vi "UHR-Fleezers Control (host) - 12.7e.vi"() -> ()   [LabVIEW 2012] (continued)
                                n2063 = local read "Delta Fl. 1"() -> (w2984:dbl)
                                n2064 = local read "Delta Fl. 2"() -> (w2982:dbl)
                                n2065 = local read "Stop All"() -> (w2991:bool)
                                n2066 = local read "APD to Watch"() -> (w2983:bool)
                                n2067 = Select(t=w2984, s=w2983, f=w2982) -> (s? t:f=w2981:dbl)
                                n2068 = Not(x=w2993) -> (.not. x?=w2992:bool)
                                n2069 = Multiply(x=w2988, y=1000.0) -> (x*y=w2987:dbl)
                                n2070 = Negate(x=w2987) -> (-x=w2986:dbl)
                                n2071 = Less?(x=w2981, y=w2986) -> (x < y?=w2990:bool)
                                n2072 = Compound Arithmetic op=OR(w2990, w2991, w2992, "Reset Force") -> (w2980:bool)
                                n2073 = case shown="True" w2980 {
                                tunnel: w2997 -> [_ w3012]
                                tunnel: w2996 -> [_ w3011]
                                tunnel: w2995 -> [_ w3001]
                                tunnel: w2994 -> [_ w3003]
                                frame False {
                                }
                                frame True {
                                n2074 = local read "Time (s)"() -> (w3002:dbl)
                                n2075 = case shown="\"Yank\"" w3011 {
                                tunnel: w3012 -> [_ w3015]
                                tunnel: w3003 -> [_ w3013]
                                frame "Image", Default {
                                }
                                frame "Yank" {
                                n2076 = flat-sequence {
                                tunnel: [w3021] -> w3016
                                tunnel: w3015 -> [w3021]
                                tunnel: [w3017] -> w3014
                                tunnel: w3013 -> [w3017]
                                tunnel: w3016 -> [w3024]
                                tunnel: w3014 -> [w3022]
                                frame #0 {
                                n2077 = local read "Yank Delay (s)"() -> (w3020:dbl)
                                n2078 = Multiply(x=w3020, y=1000.0) -> (x*y=w3018:dbl)
                                n2079 = Wait (ms)(milliseconds to wait=w3018) -> ()  [unwired: 1 out]
                                }
                                frame #1 {
                                n2080 = local read "Yank to which?"() -> (w3023:bool)
                                n2081 = case shown="False" w3023 {
                                tunnel: w3024 -> [_ w3051]
                                tunnel: w3022 -> [w3025 _]
                                frame False {
                                n2082 = flat-sequence {
                                tunnel: w3025 -> [w3026]
                                frame #0 {
                                n2083 = property on="Trap Pos FB SP" class="DigNum (strict)"("Val(Sgnl)"=w3026) -> ()  [unwired: 2 in, 2 out]
                                }
                                frame #1 {
                                n2084 = Wait (ms)(milliseconds to wait=u32 700) -> ()  [unwired: 1 out]
                                }
                                frame #2 {
                                n2085 = local read "Action (%)"() -> (w3031:dbl)
                                n2086 = Absolute Value(x=w3031) -> (abs(x)=w3030:dbl)
                                n2087 = Greater?(x=w3030, y=70.0) -> (0:w3028:bool)
                                n2088 = property on="Remove Action Offset" class="Bool (strict)"("Val(Sgnl)"=w3028) -> ()  [unwired: 2 in, 2 out]
                                }
                                frame #3 {
                                n2089 = for {
                                N: 4 -> [_]
                                n2090 = flat-sequence {
                                frame #0 {
                                n2091 = Wait (ms)(milliseconds to wait=u32 500) -> ()  [unwired: 1 out]
                                }
                                frame #1 {
                                n2092 = local read "Action (%)"() -> (w3037:dbl)
                                n2093 = Absolute Value(x=w3037) -> (abs(x)=w3036:dbl)
                                n2094 = Greater?(x=w3036, y=70.0) -> (0:w3034:bool)
                                n2095 = property on="Remove Action Offset" class="Bool (strict)"("Val(Sgnl)"=w3034) -> ()  [unwired: 2 in, 2 out]
                                }
                                }
                                }
                                }
                                frame #4 {
                                n2096 = local read "Shift confocal"() -> (w3042:bool)
                                n2097 = local read "Mean"() -> (w3044:dbl)
                                n2098 = Greater?(x=w3044, y=11.0) -> (0:w3041:bool)
                                n2099 = Not(x=w3041) -> (.not. x?=w3040:bool)
                                n2100 = And(x=w3041, y=w3042) -> (x .and. y?=w3039:bool)
                                n2101 = And(x=w3040, y=w3042) -> (x .and. y?=w3038:bool)
                                n2102 = case shown="True" w3039 {
                                frame False {
                                }
                                frame True {
                                n2103 = local read "Confocal Y 2 (V)"() -> (w3048:dbl)
                                n2104 = local read "Confocal X 2 (V)"() -> (w3047:dbl)
                                n2105 = property on="AO2" class="Slide (strict)"("Val(Sgnl)"=w3047) -> ()  [unwired: 2 in, 2 out]
                                n2106 = property on="AO1" class="Slide (strict)"("Val(Sgnl)"=w3048) -> ()  [unwired: 2 in, 2 out]
                                }
                                }
                                n2107 = case shown="True" w3038 {
                                frame False {
                                }
                                frame True {
                                n2108 = local read "Confocal X 1 (V)"() -> (w3045:dbl)
                                n2109 = local read "Confocal Y 1 (V)"() -> (w3046:dbl)
                                n2110 = property on="AO1" class="Slide (strict)"("Val(Sgnl)"=w3046) -> ()  [unwired: 2 in, 2 out]
                                n2111 = property on="AO2" class="Slide (strict)"("Val(Sgnl)"=w3045) -> ()  [unwired: 2 in, 2 out]
                                }
                                }
                                }
                                frame #5 {
                                n2112 = Wait (ms)(milliseconds to wait=u32 1500) -> ()  [unwired: 1 out]
                                }
                                frame #6 {
                                n2113 = property on="Rem fb disp offset" class="Bool (strict)"("Val(Sgnl)"=TRUE ("Value (Signaling)")) -> ()  [unwired: 2 in, 2 out]
                                }
                                }
                                }
                                frame True {
                                n2114 = flat-sequence {
                                tunnel: w3051 -> [w3052]
                                frame #0 {
                                n2115 = property on="Trap Delta (MHz)" class="DigNum (strict)"("Val(Sgnl)"=w3052) -> ()  [unwired: 2 in, 2 out]
                                }
                                frame #1 {
                                n2116 = Wait (ms)(milliseconds to wait=u32 500) -> ()  [unwired: 1 out]
                                }
                                frame #2 {
                                n2117 = local read "Shift confocal"() -> (w3058:bool)
                                n2118 = local read "Mean"() -> (w3060:dbl)
                                n2119 = Greater?(x=w3060, y=11.0) -> (0:w3057:bool)
                                n2120 = Not(x=w3057) -> (.not. x?=w3056:bool)
                                n2121 = And(x=w3057, y=w3058) -> (x .and. y?=w3055:bool)
                                n2122 = And(x=w3056, y=w3058) -> (x .and. y?=w3054:bool)
                                n2123 = case shown="True" w3055 {
                                frame False {
                                }
                                frame True {
                                n2124 = local read "Confocal Y 2 (V)"() -> (w3064:dbl)
                                n2125 = local read "Confocal X 2 (V)"() -> (w3063:dbl)
                                n2126 = property on="AO2" class="Slide (strict)"("Val(Sgnl)"=w3063) -> ()  [unwired: 2 in, 2 out]
                                n2127 = property on="AO1" class="Slide (strict)"("Val(Sgnl)"=w3064) -> ()  [unwired: 2 in, 2 out]
                                }
                                }
                                n2128 = case shown="True" w3054 {
                                frame False {
                                }
                                frame True {
                                n2129 = local read "Confocal Y 1 (V)"() -> (w3062:dbl)
                                n2130 = local read "Confocal X 1 (V)"() -> (w3061:dbl)
                                n2131 = property on="AO2" class="Slide (strict)"("Val(Sgnl)"=w3061) -> ()  [unwired: 2 in, 2 out]
                                n2132 = property on="AO1" class="Slide (strict)"("Val(Sgnl)"=w3062) -> ()  [unwired: 2 in, 2 out]
                                }
                                }
                                }
                                }
                                }
                                }
                                }
                                }
                                }
                                }
                                n2133 = local read "Messages"() -> (w3010:string)
                                n2134 = Subtract(x=w3002, y=w3001) -> (x-y=w3008:dbl)
                                "Duration (s)" <- w3008
                                n2135 = Number To Decimal String(number=w3008, width (-)=i16 0) -> (decimal integer string=w3006:string)
                                n2136 = Concatenate Strings(w3006, " s fluorescence event." ("string")) -> (w3004:string)
                                n2137 = call "Update messages.vi"("Message to add"=w3004, "Old message string"=w3010) -> ("New message string"=w3009:string)
                                n2138 = local write "Reset Force"(FALSE ("Reset Force")) -> ()
                                n2139 = local write "Waiting"(TRUE ("Waiting")) -> ()
                                n2140 = local write "Messages"(w3009) -> ()
                                n2141 = local write "Fl. High"(FALSE ("Fl. High")) -> ()
                                n2142 = call <vilib>:"Beep.vi"() -> ()  [unwired: 3 in, 9 out]
                                }
                                }
                                n2143 = node-c288() -> ()  [unwired: 2 out]
                              }
                              n2144 = node-c288(w2978) -> ()  [unwired: 1 out]
                            }
                          }
                        }
                      }
                      n2145 = local read "Trap Delta (MHz)"() -> (w2893:dbl)
                      n2146 = local read "Trap Pos FB SP"() -> (w2888:fxp<+/-,16,1>)
                    }
                  }
                }
                frame #1 {
                  n2147 = local read "Stop All"() -> (w3074:bool)
                  n2148 = local read "Fl. Triggered..."() -> (w3072:bool)
                  n2149 = Not(x=w3072) -> (.not. x?=w3073:bool)
                  n2150 = Or(x=w3073, y=w3074) -> (x .or. y?=w3071:bool)
                }
              }
              n2151 = case shown="True" w2665 {
                frame False {
                }
                frame True {
                  n2152 = local read "Confocal Y 1 (V)"() -> (w2675:dbl)
                  n2153 = local read "Confocal X 1 (V)"() -> (w2674:dbl)
                  n2154 = property on="AO2" class="Slide (strict)"("Val(Sgnl)"=w2674) -> ()  [unwired: 2 in, 2 out]
                  n2155 = property on="AO1" class="Slide (strict)"("Val(Sgnl)"=w2675) -> ()  [unwired: 2 in, 2 out]
                }
              }
              n2156 = case shown="True" w2665 {
                frame False {
                }
                frame True {
                  w2673 = FALSE ("Fl. High")
                  n2157 = local write "Waiting"(w2673) -> ()
                  n2158 = local write "Fl. High"(w2673) -> ()
                }
              }
              n2159 = node-c288() -> ()  [unwired: 2 out]
            }
            n2160 = node-c288(w2663) -> ()  [unwired: 1 out]
          }
        }
      }
      event "Stop All": Value Change {
        n2161 = event-data() -> ()  [unwired: 7 out]
        n2162 = local read "Stop All"() -> (w3079:bool)
      }
    }
    n2163 = node-c288() -> ()  [unwired: 2 out]
  }
  n2164 = timed-loop "Mouse control: trap position (AOM deflection), set confocal spot from image" {
    tunnel: [w3081] -> w74
    timing: w68 -> [_]
    timing-out: [_] -> w67
    tunnel: w5 -> [w3080]
    stop <- w3081 stop-if-true
    n2165 = node-c288() -> ()  [unwired: 2 out]
    n2166 = event shown="[0] \"Pane\": Mouse Down" {
      selector: _ -> [_ _]
      dyn-events: _ -> [_ _]
      timeout: _ -> [_ _]
      tunnel: w3080 -> [w3084 _]
      event Mouse Down {
        n2167 = event-data() -> ("Time"=w3086:u32, "Coords"=w3085:T7, "Button"=w3087:u16)  [unwired: 6 out]
        n2168 = case shown="3" w3087 {
          tunnel: w3086 -> [_ _ w3193]
          tunnel: w3085 -> [_ w3124 w3191]
          tunnel: w3084 -> [_ _ w3187]
          frame 0, Default {
          }
          frame 1 {
            n2169 = property on="APD 2" class="ImageControl"() -> ("Displayed Image Position"=w3094:cluster{"Left":i32, "Top":i32})  [unwired: 2 in, 2 out]
            n2170 = property on="APD 1" class="ImageControl"() -> ("Displayed Image Position"=w3123:cluster{"Left":i32, "Top":i32})  [unwired: 2 in, 2 out]
            n2171 = property on="Detection Laser X" class="ImageControl"() -> ("Displayed Image Position"=w3120:cluster{"Left":i32, "Top":i32})  [unwired: 2 in, 2 out]
            n2172 = property on="Detection Laser Y" class="ImageControl"() -> ("Displayed Image Position"=w3119:cluster{"Left":i32, "Top":i32})  [unwired: 2 in, 2 out]
            n2173 = property on="APD 2" class="ImageControl"() -> ("Displayed Image Size"=w3093:cluster{"Width":u32, "Height":u32})  [unwired: 2 in, 2 out]
            n2174 = property on="APD 1" class="ImageControl"() -> ("Displayed Image Size"=w3121:cluster{"Width":u32, "Height":u32})  [unwired: 2 in, 2 out]
            n2175 = property on="Detection Laser X" class="ImageControl"() -> ("Displayed Image Size"=w3122:cluster{"Width":u32, "Height":u32})  [unwired: 2 in, 2 out]
            n2176 = property on="Detection Laser Y" class="ImageControl"() -> ("Displayed Image Size"=w3118:cluster{"Width":u32, "Height":u32})  [unwired: 2 in, 2 out]
            n2177 = Unbundle By Name(w3093) -> ("Width"=w3090:u32, "Height"=w3089:u32)
            n2178 = Unbundle By Name(w3094) -> ("Left"=w3092:i32, "Top"=w3091:i32)
            n2179 = Unbundle By Name(w3121) -> ("Width"=w3115:u32, "Height"=w3114:u32)
            n2180 = Unbundle By Name(w3122) -> ("Width"=w3111:u32, "Height"=w3110:u32)
            n2181 = Unbundle By Name(w3118) -> ("Width"=w3107:u32, "Height"=w3106:u32)
            n2182 = Unbundle By Name(w3123) -> ("Left"=w3117:i32, "Top"=w3116:i32)
            n2183 = Unbundle By Name(w3120) -> ("Left"=w3113:i32, "Top"=w3112:i32)
            n2184 = Unbundle By Name(w3119) -> ("Left"=w3109:i32, "Top"=w3108:i32)
            n2185 = Bundle("Left"=w3092, "Top"=w3091, "Width"=w3090, "Height"=w3089) -> (w3088:T33)  [unwired: 1 in]
            n2186 = Bundle("Left"=w3117, "Top"=w3116, "Width"=w3115, "Height"=w3114) -> (w3105:T33)  [unwired: 1 in]
            n2187 = Bundle("Left"=w3113, "Top"=w3112, "Width"=w3111, "Height"=w3110) -> (w3104:T33)  [unwired: 1 in]
            n2188 = Bundle("Left"=w3109, "Top"=w3108, "Width"=w3107, "Height"=w3106) -> (w3103:T33)  [unwired: 1 in]
            n2189 = Build Cluster Array(w3088, w3105, w3104, w3103) -> (w3102:T34)
            n2190 = for {
              tunnel: w3124 -> [w3135]
              tunnel: w3102 -> [w3136] mode=indexing
              shift-right: [w3133] -> w3100
              shift-left: TRUE -> [w3134]
              shift-right: [w3132] -> w3098
              shift-left: _ -> [w3128]
              shift-right: [w3131] -> w3097
              shift-left: _ -> [w3127]
              shift-right: [w3130] -> w3096
              shift-left: _ -> [w3126]
              shift-right: [w3129] -> w3095
              shift-left: _ -> [w3125]
              n2191 = case shown="True" w3134 {
                selector: w3134 -> [w3141 _]
                tunnel: w3136 -> [_ w3150]
                tunnel: w3135 -> [_ w3148]
                tunnel: [w3141 w3146] -> w3133
                tunnel: [w3140 w3145] -> w3132
                tunnel: [w3139 w3144] -> w3131
                tunnel: [w3138 w3143] -> w3130
                tunnel: [w3137 w3142] -> w3129
                tunnel: w3128 -> [w3140 _]
                tunnel: w3127 -> [w3139 _]
                tunnel: w3126 -> [w3138 _]
                tunnel: w3125 -> [w3137 _]
                frame False {
                }
                frame True {
                  n2192 = Unbundle(w3150) -> (w3149:T33)
                  n2193 = call "isclickinwindow.vi"("Image Param"=w3149, "Point32"=w3148) -> ("4 Y"=w3142:i32, "3 Height"=w3143:i32, "2 X"=w3144:i32, "1 Width"=w3145:i32, "In image?"=w3147:bool)  [unwired: 1 in]
                  n2194 = Not(x=w3147) -> (.not. x?=w3146:bool)
                }
              }
            }
            n2195 = Not(x=w3100) -> (.not. x?=w3099:bool)
            n2196 = case shown="True" w3099 {
              tunnel: w3097 -> [_ w3164]
              tunnel: w3095 -> [_ w3163]
              tunnel: w3098 -> [_ w3162]
              tunnel: w3096 -> [_ w3161]
              frame False {
              }
              frame True {
                w3151 = FALSE ("Get Point")
                n2197 = local read "Scan lines (y)"() -> (w3166:u64)
                n2198 = disable-structure shown="Disabled" {
                  frame Disabled {
                  }
                  frame Enabled {
                  }
                }
                n2199 = local read "Actual MCL Inc (V)"() -> (w3160:dbl)
                n2200 = local read "Scan steps (MCL)"() -> (w3165:u64)
                n2201 = Divide "Y Pix/step"(x=w3161, y=w3166) -> (x/y=w3173:dbl)
                n2202 = Divide "Y V/pix"(x=w3160, y=w3173) -> (x/y=w3172:dbl)
                n2203 = Divide "Y half step offset"(x=w3160, y=2.0) -> (x/y=w3174:dbl)
                n2204 = Divide "X pix/step"(x=w3162, y=w3165) -> (x/y=w3171:dbl)
                n2205 = Negate(x=w3174) -> (-x=w3175:dbl)
                n2206 = local read "Initial Y"() -> (w3181:dbl)
                n2207 = Multiply(x=w3163, y=w3172) -> (x*y=w3182:dbl)
                n2208 = Divide "X half step offset"(x=w3160, y=2.0) -> (x/y=w3168:dbl)
                n2209 = Divide "X V/pix"(x=w3160, y=w3171) -> (x/y=w3170:dbl)
                n2210 = Multiply(x=w3160, y=w3165) -> (x*y=w3177:dbl)
                n2211 = Compound Arithmetic op=ADD(w3175, w3182, w3181) -> (w3152:dbl)
                "Pointer Y (V)" <- w3152
                n2212 = Multiply(x=w3170, y=w3164) -> (x*y=w3179:dbl)
                n2213 = Negate(x=w3168) -> (-x=w3167:dbl)
                n2214 = local read "Initial X"() -> (w3180:dbl)
                n2215 = Negate(x=w3179) -> (-x=w3178:dbl)
                n2216 = Compound Arithmetic op=ADD(w3167, w3177, w3180, w3178) -> (w3153:dbl)
                "Pointer X (V)" <- w3153
                n2217 = case shown="True" "Set High F Confocal Spot (X-Y)" {
                  tunnel: w3153 -> [_ w3183]
                  tunnel: w3152 -> [_ w3184]
                  frame False {
                  }
                  frame True {
                    "Confocal Y 2 (V)" <- w3184
                    "Confocal X 2 (V)" <- w3183
                  }
                }
                n2218 = Or(x="Set X Only", y="Set Confocal Spot (X-Y)") -> (x .or. y?=w3156:bool)
                n2219 = Or(x="Set Confocal Spot (X-Y)", y="Set Y Only") -> (x .or. y?=w3155:bool)
                n2220 = case shown="True" w3156 {
                  tunnel: w3153 -> [_ w3185]
                  frame False {
                  }
                  frame True {
                    n2221 = property on="AO2" class="Slide (strict)"("Val(Sgnl)"=w3185) -> ()  [unwired: 2 in, 2 out]
                    "Confocal X 1 (V)" <- w3185
                  }
                }
                n2222 = case shown="True" w3155 {
                  tunnel: w3152 -> [_ w3186]
                  frame False {
                  }
                  frame True {
                    n2223 = property on="AO1" class="Slide (strict)"("Val(Sgnl)"=w3186) -> ()  [unwired: 2 in, 2 out]
                    "Confocal Y 1 (V)" <- w3186
                  }
                }
                n2224 = local write "Set High F Confocal Spot (X-Y)"(w3151) -> ()
                n2225 = local write "Set Confocal Spot (X-Y)"(w3151) -> ()
                n2226 = local write "Set X Only"(w3151) -> ()
                n2227 = local write "Set Y Only"(w3151) -> ()
              }
            }
          }
          frame 3 {
            n2228 = local read "BD 2 Frequency 1 (MHz)"() -> (w3188:dbl)
            n2229 = local read "BD 1 Frequency 1 (MHz)"() -> (w3189:dbl)
            n2230 = local write "Manipulating Trap"(TRUE ("Manipulating Trap")) -> ()
            n2231 = local write "Coords"(T7 {"Horizontal"=0, "Vertical"=0} ("Coords")) -> ()
            n2232 = while {
              tunnel: w3193 -> [w3198]
              tunnel: w3191 -> [w3197]
              tunnel: w3189 -> [w3196]
              tunnel: w3188 -> [w3195]
              tunnel: w3187 -> [w3194]
              stop <- w3199 stop-if-true
              n2233 = event shown="[0] \"Pane\": Mouse Move" {
                selector: _ -> [_ _]
                dyn-events: _ -> [_ _]
                timeout: _ -> [_ _]
                tunnel: ["Force Manip Abort" w3263] -> w3199
                tunnel: w3198 -> [w3206 _]
                tunnel: w3197 -> [w3204 _]
                tunnel: w3196 -> [w3203 _]
                tunnel: w3195 -> [w3202 _]
                tunnel: w3194 -> [w3200 _]
                event Mouse Move {
                  n2234 = event-data() -> ("Time"=w3207:u32, "Coords"=w3208:T7)  [unwired: 3 out]
                  n2235 = Less?(x=w3207, y=w3206) -> (x < y?=w3205:bool)
                  n2236 = case "Makes sure old motion events prior to mouse click aren't used" shown="False" w3205 {
                    tunnel: w3208 -> [w3250 _]
                    tunnel: w3204 -> [w3251 _]
                    tunnel: w3203 -> [w3225 _]
                    tunnel: w3202 -> [w3224 _]
                    tunnel: w3200 -> [w3209 _]
                    frame False {
                      n2237 = Subtract(x=w3250, y=w3251) -> (x-y=w3249:T7)
                      "Coords" <- w3249
                      n2238 = local read "Y RF Frequency Limits (MHz)"() -> (w3210:T16)
                      n2239 = To Double Precision Float(number=w3249) -> (double precision float=w3248:cluster{"Horizontal":dbl, "Vertical":dbl})
                      n2240 = Multiply(x=cluster{"Horizontal":dbl, "Vertical":dbl} {"Horizontal"=-1.0, "Vertical"=1.0}, y="Manipulation Scaling") -> (x*y=w3244:cluster{"Horizontal":dbl, "Vertical":dbl})
                      n2241 = local read "X RF Frequency Limits (MHz)"() -> (w3211:T16)
                      n2242 = Multiply(x=w3248, y=w3244) -> (x*y=w3246:cluster{"Horizontal":dbl, "Vertical":dbl})
                      n2243 = Unbundle By Name(w3246) -> ("Horizontal"=w3241:dbl, "Vertical"=w3245:dbl)
                      n2244 = Unbundle By Name(w3210) -> ("Maximum"=w3213:dbl, "Minimum"=w3212:dbl)
                      n2245 = Boolean To (0,1)(Boolean="Manip. X?") -> (0, 1=w3239:i16)
                      n2246 = Boolean To (0,1)(Boolean="Manip. Y?") -> (0, 1=w3236:i16)
                      n2247 = local read "BD 1 Frequency 2 (MHz)"() -> (w3227:dbl)
                      n2248 = Multiply(x=w3245, y=w3236) -> (x*y=w3238:dbl)
                      n2249 = Multiply(x=w3239, y=w3241) -> (x*y=w3242:dbl)
                      n2250 = local read "BD 2 Frequency 2 (MHz)"() -> (w3226:dbl)
                      n2251 = Unbundle By Name(w3211) -> ("Maximum"=w3215:dbl, "Minimum"=w3214:dbl)
                      n2252 = Add(x=w3224, y=w3238) -> (x+y=w3217:dbl)
                      n2253 = Add(x=w3225, y=w3242) -> (x+y=w3219:dbl)
                      n2254 = In Range and Coerce(upper limit=w3215, x=w3219, lower limit=w3214) -> (coerced(x)=w3218:dbl)  [unwired: 1 out]
                      n2255 = In Range and Coerce(upper limit=w3213, x=w3217, lower limit=w3212) -> (coerced(x)=w3216:dbl)  [unwired: 1 out]
                      n2256 = Subtract(x=w3218, y=w3227) -> (x-y=w3235:dbl)
                      n2257 = Subtract(x=w3216, y=w3226) -> (x-y=w3234:dbl)
                      n2258 = Square(x=w3235) -> (x^2=w3233:dbl)
                      n2259 = Square(x=w3234) -> (x^2=w3232:dbl)
                      n2260 = Add(x=w3233, y=w3232) -> (x+y=w3231:dbl)
                      n2261 = Square Root(x=w3231) -> (sqrt(x)=w3228:dbl)
                      n2262 = In Range and Coerce(upper limit="Limit Max (MHz)", x=w3228, lower limit="Limit Min (MHz)") -> (In Range?=w3221:bool)  [unwired: 1 out]
                      n2263 = Not(x="Limits Enable") -> (.not. x?=w3220:bool)
                      n2264 = Or(x=w3221, y=w3220) -> (x .or. y?=w3222:bool)
                      n2265 = case shown="True" w3222 {
                        tunnel: w3228 -> [_ w3253]
                        tunnel: w3218 -> [_ w3260]
                        tunnel: w3227 -> [_ w3259]
                        tunnel: w3216 -> [_ w3258]
                        tunnel: w3226 -> [_ w3257]
                        tunnel: w3211 -> [_ w3255]
                        tunnel: w3210 -> [_ w3254]
                        tunnel: w3209 -> [_ w3252]
                        frame False {
                        }
                        frame True {
                          n2266 = local read "BD 1 Frequency 3 (MHz)"() -> (w3261:dbl)
                          n2267 = local read "BD 2 Frequency 3 (MHz)"() -> (w3256:dbl)
                          n2268 = local write "Trap Delta (MHz)"(w3253) -> ()
                          n2269 = call "set RF board frequency - interlace.vi"("Board 2 Frequency Limits"=w3254, "Board 1 Frequency Limits"=w3255, "FPGA VI Reference In"=w3252, "Board 2 Frequency 3 (MHz)"=w3256, "Board 1 Frequency 3 (MHz)"=w3261, "Board 2 Frequency 2 (MHz)"=w3257, "Board 2 Frequency 1 (MHz)"=w3258, "Board 1 Frequency 2 (MHz)"=w3259, "Board 1 Frequency 1  (MHz)"=w3260) -> ()  [unwired: 1 in, 2 out]
                          n2270 = local write "BD 2 Frequency 1 (MHz)"(w3258) -> ()
                          n2271 = local write "BD 1 Frequency 1 (MHz)"(w3260) -> ()
                        }
                      }
                    }
                    frame True {
                    }
                  }
                }
                event Mouse Up {
                  n2272 = event-data() -> ("Button"=w3262:u16)  [unwired: 8 out]
                  n2273 = case shown="3" w3262 {
                    tunnel: [FALSE TRUE] -> w3263
                    frame 0, Default {
                    }
                    frame 3 {
                      n2274 = local read "Trap Delta (MHz)"() -> (w3265:dbl)
                      n2275 = property on="Initial delta (MHz)" class="DigNum (strict)"("Val(Sgnl)"=w3265) -> ()  [unwired: 2 in, 2 out]
                      n2276 = local write "Manipulating Trap"(FALSE ("Manipulating Trap")) -> ()
                    }
                  }
                }
              }
            }
          }
        }
      }
      event Mouse Move {
        n2277 = event-data() -> ()  [unwired: 6 out]
      }
    }
    n2278 = local read "Stop All"() -> (w3081:bool)
    n2279 = node-c288() -> ()  [unwired: 2 out]
  }
  n2280 = flat-sequence "Video" {
    tunnel: [w3277] -> w55
    tunnel: w55 -> [w3317]
    frame #0 {
      n2281 = while {
        stop <- w3269 continue-if-true
        n2282 = call "Close Video Capture.vi"() -> ("error code OUT"=w3271:i32)
        n2283 = Equal?(x=w3271, y=0) -> (x = y?=w3269:bool)
      }
      n2284 = local write "Stop All"(FALSE ("Stop All")) -> ()
    }
    frame #1 {
      n2285 = call "DMR_Init.vi"() -> ()  [unwired: 3 out]
    }
    frame #2 {
      w3272 = "DE245428202"  # MSU fleezers card #
      (unwired) "DE019116701"  # Illinois fleezers card #
      # "Setting the destination format to Mono8 makes sure that the image can be displayed in the intensity plot."
      n2286 = call "DMR_GetDevice.vi"("search string IN"=w3272) -> ("device handle OUT"=w3295:i32)  [unwired: 4 in, 2 out]
      n2287 = call "DMR_OpenDevice.vi"("device handle IN"=w3295) -> ("driver handle OUT"=w3278:i32)  [unwired: 4 out]
      n2288 = call "DMR_FindList.vi"("flags IN"=u32 0 ("flags"), "list name IN"="" ("String"), "list type IN"=T35."camera descriptions", "driver handle IN"=w3278) -> ("list handle OUT"=w3281:i32)  [unwired: 2 out]
      n2289 = call "DMR_FindList.vi"("flags IN"=u32 0 ("flags"), "list name IN"="Base", "list type IN"=T35."setting", "driver handle IN"=w3278) -> ("list handle OUT"=w3279:i32)  [unwired: 2 out]
      n2290 = call "OBJ_GetHandle.vi"("object name IN"="VideoStandard", "list handle IN"=w3281) -> ("object handle OUT"=w3275:i32)  [unwired: 3 out]
      n2291 = call "OBJ_GetHandle.vi"("object name IN"="PixelFormat", "list handle IN"=w3279) -> ("object handle OUT"=w3289:i32)  [unwired: 3 out]
      n2292 = call "OBJ_SetS.vi"("value index IN"=0, "value IN"="NTSC M", "object handle IN"=w3275) -> ()  [unwired: 2 out]
      n2293 = call "OBJ_SetS.vi"("value index IN"=0, "value IN"="Mono8" ("value"), "object handle IN"=w3289) -> ()  [unwired: 2 out]
      n2294 = call "OBJ_GetHandle.vi"("object name IN"="VideoChannel", "list handle IN"=w3279) -> ("object handle OUT"=w3285:i32)  [unwired: 3 out]
      n2295 = while {
        tunnel: [w3299] -> w3277
        tunnel: w3278 -> [w3296]
        stop <- w3297 continue-if-true
        n2296 = call "DMR_ImageRequestSingle.vi"("request control IN"=0, "driver handle IN"=w3296) -> ("error code OUT"=w3298:i32, "driver handle OUT"=w3299:i32)  [unwired: 2 out]
        n2297 = Equal To 0?(x=w3298) -> (x = 0?=w3297:bool)
      }
      n2298 = call "OBJ_SetI.vi"("value index IN"=0, "value IN"=3 ("Video channel"), "object handle IN"=w3285) -> ()  [unwired: 2 out]
    }
    frame #3 {
      w3305 = T19 0 items=["Grayscale (U8)", "Grayscale (I16)", "Grayscale (SGL)", "Complex (CSG)", "RGB (U32)", "HSL (U32)", "RGB (U64)"] ("Image Type")
      w3313 = T19 0 items=["Grayscale (U8)", "Grayscale (I16)", "Grayscale (SGL)", "Complex (CSG)", "RGB (U32)", "HSL (U32)", "RGB (U64)"] ("Image Type")
      n2299 = for "Create Greyscale map" {
        N: 256 -> [_]
        tunnel: [w3319] -> w3302 mode=indexing
        workers-P: _ -> [_]
        i -> [w3322]
        n2300 = To Unsigned Byte Integer(number=w3322) -> (unsigned 8bit integer=w3318:u8)
        n2301 = Join Numbers(hi=w3318, lo=w3318) -> ((hi.lo)=w3321:u16)
        n2302 = Join Numbers(hi=w3318, lo=w3318) -> ((hi.lo)=w3320:u16)
        n2303 = Join Numbers(hi=w3321, lo=w3320) -> ((hi.lo)=w3319:u32)
      }
      n2304 = call "IMAQ Create"("Image Name"="Scaled video", "Image Type"=w3305) -> ("New Image"=w3304:T2)  [unwired: 2 in, 2 out]
      n2305 = call "IMAQ Create"("Image Name"="Main video", "Image Type"=w3313) -> ("New Image"=w3314:T2)  [unwired: 2 in, 2 out]
      n2306 = node-c288(0 ("Processor")) -> (w3312:T23)  [unwired: 3 out]
      n2307 = Initialize Array(u32 0 ("Window Number (0...15)"), 480 ("dimension size"), 640 ("dimension size")) -> (w3307:u32[][])
      n2308 = timed-loop {
        tunnel: w3317 -> [w3339]
        tunnel: [w3338] -> w3316
        tunnel: w3314 -> [w3337]
        timing: w3312 -> [_]
        timing-out: [_] -> w3311
        tunnel: w3307 -> [w3326]
        tunnel: w3304 -> [w3324]
        tunnel: w3302 -> [w3323]
        stop <- w3325 stop-if-true
        # "This block performs the \nactual image capture."
        n2309 = node-c288() -> ()  [unwired: 2 out]
        n2310 = local read "Stop All"() -> (w3325:bool)
        n2311 = Reciprocal(x="Video Capture Rate (Hz)") -> (1/x=w3329:dbl)
        n2312 = Multiply(x=w3329, y=1000.0) -> (x*y=w3327:dbl)
        n2313 = call "DMR_ImageRequestWaitFor.vi"("queue number IN"=0, "timeout(ms) IN"=500, "driver handle IN"=w3339) -> ("error code OUT"=w3343:i32, "request number OUT"=w3340:i32, "driver handle OUT"=w3341:i32)
        n2314 = feedback #1(T36 refnum ("Avi Refnum")) -> (w3331:T36)
        n2315 = case shown="True" "New Video File" {
          tunnel: [T36 refnum ("Avi Refnum") w3360] -> w3333
          tunnel: [FALSE TRUE] -> w3334
          tunnel: w3331 -> [_ w3356]
          frame False {
          }
          frame True {
            n2316 = call "Create new save file.vi"("Ext"=".avi" ("string"), "Index In"="Video Index") -> ("Path Out"=w3352:path, "Index Out"=w3353:dbl)  [unwired: 1 in]
            "Path Out" <- w3352
            n2317 = Not Equal?(x=w3356, y=T36 refnum ("Avi Refnum")) -> (x != y?=w3357:bool)
            n2318 = Increment(x=w3353) -> (x+1=w3362:dbl)
            n2319 = case shown="True" w3357 {
              tunnel: w3356 -> [_ w3363]
              frame False {
              }
              frame True {
                n2320 = call "IMAQ AVI Close"("Avi Refnum"=w3363) -> ()  [unwired: 1 in, 10 out]
              }
            }
            n2321 = local write "Video Index"(w3362) -> ()
            n2322 = call "IMAQ AVI Create"("Frames Per Second"=u32 30, "AVI Path"=w3352) -> ("Avi Refnum"=w3360:T36)  [unwired: 5 in, 4 out]
          }
        }
        n2323 = Equal To 0?(x=w3343) -> (x = 0?=w3342:bool)
        n2324 = Select(t=w3333, s=w3334, f=w3331) -> (s? t:f=w3332:T36)
        n2325 = feedback-in #1(w3332) -> ()
        n2326 = case shown="True" w3342 {
          tunnel: w3341 -> [w3364 w3398]
          tunnel: w3340 -> [_ w3397]
          tunnel: [w3364 w3394] -> w3338
          tunnel: w3337 -> [_ w3379]
          tunnel: w3326 -> [_ w3383]
          tunnel: w3332 -> [_ w3381]
          tunnel: w3324 -> [_ w3376]
          tunnel: w3323 -> [_ w3375]
          frame False {
          }
          frame True {
            w3388 = u32 0 ("X-offset IN")
            n2327 = call "DMR_GetImageRequestBufferData.vi"("driver handle IN"=w3398, "request number IN"=w3397) -> ("width OUT"=w3387:i32, "height OUT"=w3386:i32, "driver handle OUT"=w3393:i32, "request number OUT"=w3392:i32, "bytes per pixel OUT"=w3389:i32)  [unwired: 13 out]
            n2328 = call "DMR_GetImageRequestBufferImageData.vi"("driver handle IN"=w3393, "request number IN"=w3392, "bytes per pixel IN"=w3389, "X-offset IN"=w3388, "Y-offset IN"=w3388, "height IN"=w3386, "width IN"=w3387) -> ("driver handle OUT"=w3391:u32, "request number OUT"=w3390:u32, "image OUT"=w3368:u32[][])  [unwired: 10 out]
            n2329 = Transpose 2D Array(2D array=w3368) -> (transposed array=w3374:u32[][])
            n2330 = Select(t=w3374, s="Flip Y (or X)", f=w3368) -> (s? t:f=w3373:u32[][])
            n2331 = call "DMR_ImageRequestUnlock.vi"("request number IN"=w3390, "driver handle IN"=w3391) -> ("driver handle OUT"=w3396:i32)  [unwired: 1 in, 2 out]
            n2332 = for {
              tunnel: w3373 -> [w3433] mode=indexing
              tunnel: [w3432] -> w3371 mode=indexing
              n2333 = Reverse 1D Array(array=w3433) -> (reversed array=w3432:u32[])
            }
            n2334 = call "DMR_ImageRequestSingle.vi"("request control IN"=0, "driver handle IN"=w3396) -> ("driver handle OUT"=w3394:i32)  [unwired: 3 out]
            n2335 = Transpose 2D Array(2D array=w3371) -> (transposed array=w3372:u32[][])
            n2336 = Select(t=w3372, s="Flip Y (or X)", f=w3371) -> (s? t:f=w3369:u32[][])
            n2337 = Select(t=w3369, s="Flip Image", f=w3368) -> (s? t:f=w3366:u32[][])
            n2338 = case shown="True" "Averaging" {
              tunnel: w3366 -> [w3436 w3441]
              tunnel: [w3436 w3440] -> w3380
              tunnel: w3383 -> [_ w3438]
              frame False {
              }
              frame True {
                (unwired) 1
                w3446 = 1
                n2339 = feedback #2(w3438) -> (w3437:u32[][])
                n2340 = Add(x=w3441, y=w3437) -> (x+y=w3442:u32[][])
                n2341 = Select(t=w3438, s="Reset Averaging", f=w3442) -> (s? t:f=w3444:u32[][])
                n2342 = feedback-in #2(w3444) -> ()
                n2343 = feedback #3(w3446) -> (w3439:i32)
                n2344 = Divide(x=w3442, y=w3439) -> (x/y=w3443:dbl[][])
                n2345 = Increment(x=w3439) -> (x+1=w3447:i32)
                n2346 = To Unsigned Long Integer(number=w3443) -> (unsigned 32bit integer=w3440:u32[][])
                n2347 = Select(t=w3446, s="Reset Averaging", f=w3447) -> (s? t:f=w3445:i32)
                n2348 = feedback-in #3(w3445) -> ()
              }
            }
            n2349 = case shown="True" "Zoom video window" {
              tunnel: w3380 -> [_ w3412]
              tunnel: w3376 -> [_ w3411]
              frame False {
              }
              frame True {
                n2350 = To Double Precision Float(number=w3412) -> (double precision float=w3409:dbl[][])
                n2351 = In Range and Coerce(upper limit="Intensity Upper", x=w3409, lower limit="Intensity Lower") -> (coerced(x)=w3408:dbl[][])  [unwired: 1 out]
                n2352 = Subtract(x="Intensity Upper", y="Intensity Lower") -> (x-y=w3405:dbl)
                n2353 = Subtract(x=w3408, y="Intensity Lower") -> (x-y=w3406:dbl[][])
                n2354 = Divide(x=w3406, y=w3405) -> (x/y=w3407:dbl[][])
                n2355 = Multiply(x=255.0, y=w3407) -> (x*y=w3403:dbl[][])
                n2356 = To Unsigned Byte Integer(number=w3403) -> (unsigned 8bit integer=w3410:u8[][])
                n2357 = call "IMAQ ArrayToImage"("Image Pixels (U8)"=w3410, "Image"=w3411) -> ("Image Out"=w3399:T2)  [unwired: 4 in, 5 out]
                n2358 = First Call?() -> (First Call?: T/F=w3400:bool)
                n2359 = case shown="True" w3400 {
                  tunnel: w3399 -> [w3413 w3424]
                  frame False {
                    n2360 = flat-sequence {
                      tunnel: w3413 -> [w3419]
                      frame #0 {
                        w3416 = FALSE ("Get/Set Status? (Set)")
                        w3415 = 0 ("Window Number (0...15)")
                        n2361 = call "IMAQ WindSize"("Get/Set Status? (Set)"=w3416, "Window Number"=w3415) -> ("Width & Height out"=→"Window Size":cluster{"Width":i32, "Height":i32})  [unwired: 4 in, 2 out]
                        n2362 = call "IMAQ WindMove"("Window Number (0...15)"=w3415, "Get/Set Status? (Set)"=w3416) -> ("Coordinates (screen)"=→"Window Position":cluster{"X Position":i32, "Y Position":i32})  [unwired: 3 in, 1 out]
                        n2363 = call "IMAQ WindDraw"("Resize to Image Size? (Y)"=FALSE, "Window Number (0...15)"=w3415, "Image"=w3419) -> ()  [unwired: 7 in, 2 out]
                      }
                      frame #1 {
                        n2364 = call "IMAQ WindZoom 2"("Center Point"="Center Point", "Zoom to Fit? (False)"=FALSE, "Zoom Factor"="Zoom Factor") -> ()  [unwired: 5 in, 4 out]
                      }
                    }
                  }
                  frame True {
                    n2365 = flat-sequence {
                      tunnel: w3424 -> [w3427]
                      tunnel: [w3425] -> w3423
                      tunnel: w3423 -> [w3429]
                      frame #0 {
                        w3426 = TRUE ("Resize to Image Size? (Y)")
                        w3425 = 0 ("Window Number (0...15)")
                        n2366 = call "IMAQ WindNonTearing"("Window Number"=w3425, "NonTearing? (True)"=w3426) -> ()  [unwired: 8 in, 2 out]
                        n2367 = call "IMAQ WindDraw"("Resize to Image Size? (Y)"=w3426, "Window Number (0...15)"=w3425, "Image"=w3427) -> ()  [unwired: 7 in, 2 out]
                      }
                      frame #1 {
                        n2368 = call "IMAQ WindSize"("Scrollbars? (N)"=FALSE, "Width & Height"="Initial Window Size", "Window Number"=w3429) -> ()  [unwired: 3 in, 3 out]
                        n2369 = call "IMAQ WindMove"("Window Number (0...15)"=w3429, "Coordinates (screen)"="Initial Window Position") -> ()  [unwired: 3 in, 2 out]
                      }
                    }
                  }
                }
              }
            }
            n2370 = To Unsigned Byte Integer(number=w3380) -> (unsigned 8bit integer=w3378:u8[][])
            n2371 = call "IMAQ ArrayToImage"("Image Pixels (U8)"=w3378, "Image"=w3379) -> ("Image Out"=w3377:T2)  [unwired: 4 in, 5 out]
            "Primary Video Display" <- w3377
            n2372 = case shown="True" "Save Video" {
              tunnel: w3381 -> [_ w3435]
              tunnel: w3377 -> [_ w3434]
              frame False {
              }
              frame True {
                n2373 = call "IMAQ AVI Write Frame"("Image"=w3434, "Avi Refnum"=w3435) -> ()  [unwired: 2 in, 8 out]
              }
            }
            n2374 = case shown="True" "Save Image" {
              tunnel: w3378 -> [_ w3450]
              tunnel: w3375 -> [_ w3449]
              frame False {
              }
              frame True {
                n2375 = call <vilib>:"Flatten Pixmap.vi"("colors"=w3449, "8-bit pixmap"=w3450) -> ("image data"=w3456:T37)  [unwired: 4 in, 5 out]
                n2376 = call "Create new save file.vi"("Insert"="video_frame_" ("string"), "Ext"=".bmp" ("string"), "Index In"="Image Index") -> ("Path Out"=w3452:path, "Index Out"=w3457:dbl)
                n2377 = Increment(x=w3457) -> (x+1=w3451:dbl)
                n2378 = local write "Image Index"(w3451) -> ()
                n2379 = call <vilib>:"Write BMP File.vi"("image data"=w3456, "path to BMP file"=w3452) -> ()  [unwired: 1 in, 9 out]
              }
            }
          }
        }
        n2380 = node-c288(w3327) -> ()  [unwired: 1 out]
      }
      n2381 = node-c288(w3311) -> ()  [unwired: 1 out]
      n2382 = call "DMR_CloseDevice.vi"("driver handle IN"=w3316) -> ()  [unwired: 1 in, 4 out]
    }
    frame #4 {
      n2383 = call "DMR_Close.vi"() -> ()  [unwired: 1 out]
    }
  }
  n2384 = node-c288(i64 1 ("Period"), 1 ("Processor")) -> (w73:T23)  [unwired: 2 out]
  n2385 = timed-loop "Main data acquisition loop (get data, process data for display, and save data to disk)" {
    tunnel: w11 -> [w3780]
    tunnel: w10 -> [w3779]
    tunnel: [w3808] -> w80
    tunnel: [w3803] -> w79
    timing: w73 -> [_]
    timing-out: [_] -> w72
    tunnel: w47 -> [w3634]
    stop <- "Stop All" stop-if-true
    w3551 = "Initialize"
    # "T2 sum"
    # "T1 sum"
    # "Fluorescence data into FIFO for external control vi's\n(e.g., fluorescence triggering) - Duncan Nall"
    n2386 = node-c288() -> ()  [unwired: 2 out]
    n2387 = First Call?() -> (First Call?: T/F=w3586:bool)
    n2388 = Or(x="Reset", y=w3586) -> (x .or. y?=w3587:bool)
    n2389 = local read "Flushing P1"() -> (w3506:bool)
    n2390 = case "Reset data stream (manual reset or at begining of some rastering and imaging)" shown="True" w3587 {
      tunnel: w3780 -> [w4849 w4857]
      tunnel: w3779 -> [w4848 w4856]
      tunnel: [w4849 w4851] -> w3775
      tunnel: [w4848 w4850] -> w3774
      frame False {
      }
      frame True {
        w4854 = TRUE ("AI to FIFO")
        n2391 = local write "Overflow (data lost)"(FALSE ("Overflow (data lost)")) -> ()
        n2392 = call "reset FPGA DMA.vi"("error in"=w4856, "FPGA VI Reference In"=w4857) -> ("error out"=w4852:errorcluster, "FPGA VI Reference Out"=w4853:T20)
        n2393 = xnode "Read/Write Control"("FPGA VI Reference In"=w4853, "error in"=w4852, "AI to FIFO"=w4854, "APD to FIFO"=w4854) -> ("FPGA VI Reference Out"=w4851:T20, "error out"=w4850:errorcluster)
      }
    }
    n2394 = case shown="True" w3506 {
      frame False {
      }
      frame True {
        n2395 = local read "Flush rate (uL/m) P1"() -> (w3838:dbl)
        n2396 = local read "HP1 Flush Time (s)"() -> (w3847:dbl)
        n2397 = local read "DMA Update Period (s)"() -> (w3841:dbl)
        n2398 = Divide(x=w3838, y=60.0) -> (x/y=w3839:dbl)
        n2399 = Divide(x=w3847, y=w3841) -> (x/y=w3836:dbl)
        n2400 = feedback #4(0) -> (w3845:i32)
        n2401 = Increment(x=w3845) -> (x+1=w3835:i32)
        n2402 = Greater?(x=w3835, y=w3836) -> (0:w3844:bool)
        n2403 = Compound Arithmetic op=MULTIPLY(w3841, w3835, w3839) -> (→"P1 Flush Volume (uL)":dbl)
        n2404 = Divide(x=w3835, y=w3836) -> (x/y=→"P1 Flushing Bar":dbl)
        n2405 = case shown="True" w3844 {
          tunnel: w3835 -> [w3848 _]
          tunnel: [w3848 0] -> w3843
          frame False {
          }
          frame True {
            w3849 = FALSE ("Flushing P1")
            n2406 = local write "Inject Pump 1"(w3849) -> ()
            n2407 = local write "Flushing P1"(w3849) -> ()
            n2408 = property on="Clear Volume P1" class="Bool (strict)"("Val(Sgnl)"=TRUE ("Value (Signaling)")) -> ()  [unwired: 2 in, 2 out]
          }
        }
        n2409 = feedback-in #4(w3843) -> ()
      }
    }
    n2410 = Or(x="Start AOD Scan", y="Trap Raster Scan") -> (x .or. y?=w3731:bool)
    n2411 = case "Start AOM raster scan" shown="True" w3731 {
      tunnel: w3775 -> [w4699 w4709]
      tunnel: w3774 -> [w4698 w4708]
      tunnel: [w4699 w4702] -> w3773
      tunnel: [w4698 w4701] -> w3772
      frame False {
      }
      frame True {
        n2412 = case shown="True" "Restart DMA? (AOD)" {
          tunnel: [w4747 w4749] -> w4703
          tunnel: [w4746 w4748] -> w4704
          tunnel: w4709 -> [w4747 w4751]
          tunnel: w4708 -> [w4746 w4750]
          frame False {
          }
          frame True {
            n2413 = local write "Overflow (data lost)"(FALSE ("Overflow (data lost)")) -> ()
            n2414 = call "reset FPGA DMA.vi"("error in"=w4750, "FPGA VI Reference In"=w4751) -> ("error out"=w4748:errorcluster, "FPGA VI Reference Out"=w4749:T20)
          }
        }
        n2415 = local write "Trap Raster Scan"(FALSE ("Trap Raster Scan")) -> ()
        n2416 = case shown="True" "Move MCL Also?" {
          tunnel: w4704 -> [w4712 w4741]
          tunnel: w4703 -> [w4713 w4742]
          tunnel: [w4711 w4745] -> w4702
          tunnel: [w4710 w4744] -> w4701
          frame False {
            w4714 = TRUE ("AI to FIFO")
            n2417 = xnode "Read/Write Control"("FPGA VI Reference In"=w4713, "error in"=w4712, "AI to FIFO"=w4714, "APD to FIFO"=w4714, "Start scan"=w4714) -> ("FPGA VI Reference Out"=w4711:T20, "error out"=w4710:errorcluster)
          }
          frame True {
            w4738 = FALSE ("1D or 2D Scan?")
            w4743 = TRUE ("AI to FIFO")
            # "Count for MCL loop"
            # "N total cycles"
            # "N steps"
            # "V_int"
            n2418 = local read "Scan Range (nm)"() -> (w4720:dbl)
            n2419 = local read "Number of F/B Scans (AOD)"() -> (w4737:u16)
            n2420 = Sign(1:w4720) -> (0:w4719:dbl)
            n2421 = Compound Arithmetic op=MULTIPLY(w4720, "MCL Step Position Ratio", "MCL/AOM Scale Tweak") -> (w4724:dbl)
            n2422 = Negate(x=w4719) -> (-x=w4716:dbl)
            n2423 = Multiply(x=w4716, y="MCL Step Increment (V_int)") -> (x*y=w4718:dbl)
            n2424 = Divide(x=w4724, y="MCL X Cal (nm/V)") -> (x/y=w4730:dbl)
            n2425 = Multiply(x=32767.0 ("y"), y=w4730) -> (x*y=w4736:dbl)
            n2426 = local read "Total Counts (ticks)"() -> (w4721:u16)
            n2427 = local read "Cycles/step (AOD)"() -> (w4732:u64)
            n2428 = local read "Scan steps (AOD)"() -> (w4733:u64)
            n2429 = Divide(x=w4736, y=10.0) -> (x/y=w4729:dbl)
            n2430 = Divide(x=w4729, y="MCL Step Increment (V_int)") -> (x/y=w4727:dbl)
            n2431 = Absolute Value(x=w4727) -> (abs(x)=w4715:dbl)
            n2432 = Compound Arithmetic op=MULTIPLY(w4733, w4732, w4721) -> (w4728:u64)
            n2433 = local write "wait to reset values"(w4743) -> ()
            n2434 = local write "MCL Scanning"(w4743) -> ()
            n2435 = Divide(x=w4728, y=w4715) -> (x/y=w4725:dbl)
            "MCL Count" <- w4725
            n2436 = xnode "Read/Write Control"("FPGA VI Reference In"=w4742, "error in"=w4741, "Scan steps (MCL)"=w4715, "Number of scans (MCL)"=w4737, "Cycles per step (MCL)"=u64 1, "Scan freq.  increment (MCL)"=w4718, "1D or 2D Scan?"=w4738, "MCL Scan Axis"=w4738, "Cont. Scan (MCL)"=w4738, "MCL count"=w4725) -> ("FPGA VI Reference Out"=w4740:T20, "error out"=w4739:errorcluster)
            n2437 = xnode "Read/Write Control"("FPGA VI Reference In"=w4740, "error in"=w4739, "AI to FIFO"=w4743, "APD to FIFO"=w4743, "Start scan"=w4743, "Start scan (MCL)"=w4743) -> ("FPGA VI Reference Out"=w4745:T20, "error out"=w4744:errorcluster)
          }
        }
        "Raster Scanning..." <- TRUE ("Scanning...")
      }
    }
    n2438 = local read "Flushing P3"() -> (w3507:bool)
    n2439 = case "Keep track of when Harvard Pump 3 is done flushing" shown="True" w3507 {
      frame False {
      }
      frame True {
        n2440 = local read "Flush rate (uL/m) P3"() -> (w3855:dbl)
        n2441 = local read "DMA Update Period (s)"() -> (w3857:dbl)
        n2442 = local read "HP3 Flush Time (s)"() -> (w3864:dbl)
        n2443 = Divide(x=w3855, y=60.0) -> (x/y=w3853:dbl)
        n2444 = feedback #5(0) -> (w3862:i32)
        n2445 = Increment(x=w3862) -> (x+1=w3856:i32)
        n2446 = Divide(x=w3864, y=w3857) -> (x/y=w3858:dbl)
        n2447 = Greater?(x=w3856, y=w3858) -> (0:w3861:bool)
        n2448 = Compound Arithmetic op=MULTIPLY(w3857, w3856, w3853) -> (→"P3 Flush Volume (uL)":dbl)
        n2449 = case shown="True" w3861 {
          tunnel: w3856 -> [w3865 _]
          tunnel: [w3865 0] -> w3860
          frame False {
          }
          frame True {
            w3866 = FALSE ("Flushing P3")
            n2450 = local write "Inject Pump 3"(w3866) -> ()
            n2451 = local write "Flushing P3"(w3866) -> ()
            n2452 = property on="Clear Volume P3" class="Bool (strict)"("Val(Sgnl)"=TRUE ("Value (Signaling)")) -> ()  [unwired: 2 in, 2 out]
          }
        }
        n2453 = feedback-in #5(w3860) -> ()
        n2454 = Divide(x=w3856, y=w3858) -> (x/y=→"P3 Flushing Bar":dbl)
      }
    }
    n2455 = And(x="Save scans", y=w3731) -> (x .and. y?=w3771:bool)
    n2456 = Compound Arithmetic op=OR("Start MCL Scan", "Confocal Image", "Confocal Linescan") -> (w3729:bool)
    n2457 = And(x="Save Data (MCL)", y=w3729) -> (x .and. y?=w3770:bool)
    n2458 = case "Start MCL raster scan" shown="True" w3729 {
      tunnel: w3773 -> [w4311 w4327]
      tunnel: w3772 -> [w4310 w4326]
      tunnel: [w4311 w4322] -> w3633
      tunnel: [w4310 w4321] -> w3632
      tunnel: [FALSE w4320] -> w3756
      tunnel: "Start MCL Scan" -> [_ w4315]
      tunnel: "Confocal Image" -> [_ w4314]
      tunnel: "Confocal Linescan" -> [_ _]
      frame False {
      }
      frame True {
        w4320 = TRUE
        n2459 = case shown="True" "Restart DMA? (MCL)" {
          tunnel: [w4372 w4374] -> w4325
          tunnel: [w4371 w4373] -> w4324
          tunnel: w4327 -> [w4372 w4377]
          tunnel: w4326 -> [w4371 w4376]
          frame False {
          }
          frame True {
            n2460 = call "reset FPGA DMA.vi"("error in"=w4376, "FPGA VI Reference In"=w4377) -> ("error out"=w4373:errorcluster, "FPGA VI Reference Out"=w4374:T20)
            n2461 = local write "Overflow (data lost)"(FALSE ("Overflow (data lost)")) -> ()
          }
        }
        n2462 = case shown="False" w4315 {
          selector: w4315 -> [_ w4331]
          tunnel: w4314 -> [w4330 _]
          tunnel: [w4330 w4331] -> w4313
          frame False {
            n2463 = property on="2D or 1D Scan" class="Bool (strict)"("Val(Sgnl)"=w4330) -> ()  [unwired: 2 in, 2 out]
            n2464 = property on="Confocal Image" class="Bool (strict)"("Value"=FALSE ("Start Confocal Map")) -> ()  [unwired: 2 in, 2 out]
          }
          frame True {
          }
        }
        n2465 = local write "MCL Scanning"(w4320) -> ()
        n2466 = local read "AO1"() -> (w4317:dbl)
        n2467 = local read "AO2"() -> (w4316:dbl)
        n2468 = case shown="True" "Center Scan" {